vi "AeroQuadConfigurator.vi"() -> ()   [LabVIEW 2009] (continued)
                  n217 = local write "DerivativePitchLevel"(w359) -> ()
                }
                frame #5 {
                  n218 = Index Array(array=w365) -> (element #1=w367:dbl, element #2=w366:dbl)  [unwired: 2 in]
                  n219 = local write "Level Limit"(w367) -> ()
                  n220 = local write "Level Off"(w366) -> ()
                }
                frame #6 {
                  n221 = Index Array(array=w374) -> (element #1=w373:dbl, element #2=w372:dbl, element #3=w371:dbl, element #4=w370:dbl, element #5=w369:dbl, element #6=w368:dbl)  [unwired: 6 in]
                  n222 = local write "Roll Smoothing"(w373) -> ()
                  n223 = local write "Pitch Smoothing"(w372) -> ()
                  n224 = local write "Yaw  Smoothing"(w371) -> ()
                  n225 = local write "Throttle Smoothing"(w370) -> ()
                  n226 = local write "Mode  Smoothing"(w369) -> ()
                  n227 = local write "Aux  Smoothing"(w368) -> ()
                }
              }
            }
            n228 = local write "Status"("Reading Configuration" ("Connection Status")) -> ()
            n229 = Bundle By Name(cluster=w320, "Error"=w311) -> (w321:T11)
          }
        }
      }
      frame #18 {
        n230 = Unbundle By Name(w378) -> ("Connected"=w376:bool, "COMport"=w379:refnum<visa-resource-name>)
        n231 = case shown="True" w376 {
          tunnel: w379 -> [_ w392]
          tunnel: w378 -> [w380 w390]
          tunnel: [w380 w389] -> w377
          tunnel: w375 -> [_ w385]
          frame #0 {
          }
          frame #1 {
            n232 = Flush Queue(queue=w385) -> (queue out=w387:refnum<queue>)  [unwired: 1 in, 2 out]
            n233 = property on="PID / Sensor Output" class="WFChart (strict)"("History Data"=cluster{"[0]":i16, "[1]":i16, "[2]":i16}[] []) -> ()  [unwired: 2 in, 2 out]
            n234 = VISA Write(VISA resource name=w392, write buffer="S") -> (error out=w388:errorcluster)  [unwired: 1 in, 2 out]
            n235 = Bundle By Name(cluster=w390, "Error"=w388) -> (w389:T11)
            n236 = property on="Motor Commands" class="WFChart (strict)"("History Data"=T9 []) -> ()  [unwired: 2 in, 2 out]
            n237 = Enqueue Element(queue=w387, element="Read AeroQuad Data") -> (queue out=w384:refnum<queue>)  [unwired: 1 in, 3 out]
            n238 = Enqueue Element(queue=w384, element="Status:Reading Flight Data") -> ()  [unwired: 1 in, 4 out]
          }
        }
      }
      frame #19 {
        n239 = Unbundle By Name(w405) -> ("Connected"=w402:bool, "COMport"=w406:refnum<visa-resource-name>, "Timeout"=w393:u32)
        n240 = Spreadsheet String To Array(delimiter (Tab)=",", format string="%s", spreadsheet string=w400, array type (2D Dbl)=string[] []) -> (array=w396:string[])
        n241 = Build Array (concatenate)("a0;", w396) -> (w394:string[])
        n242 = case shown="True" w402 {
          tunnel: w406 -> [_ w412]
          tunnel: [w409 w415] -> w404
          tunnel: w394 -> [_ w414]
          tunnel: w401 -> [w408 _]
          tunnel: w393 -> [_ w410]
          frame #0 {
            n243 = local write "Status"("Not Connected to AeroQuad" ("Connection Status")) -> ()
            n244 = Flush Queue(queue=w408) -> (error out=w409:errorcluster)  [unwired: 1 in, 2 out]
          }
          frame #1 {
            n245 = property class="Instr"(reference=w412, "Timeout"=w410) -> (reference out=w413:refnum<visa-resource-name>, error out=w411:errorcluster)  [unwired: 1 in]
            n246 = VISA Write(VISA resource name=w413, write buffer="X", error in (no error)=w411) -> (VISA resource name out=w418:refnum<visa-resource-name>, error out=w420:errorcluster)  [unwired: 1 out]
            n247 = call "Time Delay18"("error in (no error)"=w420) -> ("error out"=w419:errorcluster)  [unwired: 1 in, 9 out]
            n248 = VISA Flush I/O Buffer(VISA resource name=w418, error in (no error)=w419) -> (VISA resource name out=w416:refnum<visa-resource-name>, error out=w417:errorcluster)  [unwired: 1 in]
            n249 = for {
              tunnel: w416 -> [w424]
              shift-right: [w423] -> w415
              shift-left: w417 -> [w425]
              tunnel: w414 -> [w422] mode=indexing
              n250 = VISA Write(VISA resource name=w424, write buffer=w422, error in (no error)=w425) -> (error out=w423:errorcluster)  [unwired: 2 out]
            }
          }
        }
        n251 = Bundle By Name(cluster=w405, "Error"=w404) -> (w403:T11)
      }
      frame #20 {
        n252 = Unbundle By Name(w431) -> ("Connected"=w428:bool, "COMport"=w432:refnum<visa-resource-name>)
        n253 = case shown="True" w428 {
          tunnel: w432 -> [_ w448]
          tunnel: [w435 w439] -> w430
          tunnel: w426 -> [_ w437]
          tunnel: w427 -> [w434 w445]
          frame #0 {
            n254 = local write "Status"("Not Connected to AeroQuad" ("Connection Status")) -> ()
            n255 = Flush Queue(queue=w434) -> (error out=w435:errorcluster)  [unwired: 1 in, 2 out]
          }
          frame #1 {
            n256 = VISA Write(VISA resource name=w448, write buffer="X") -> (VISA resource name out=w449:refnum<visa-resource-name>, error out=w451:errorcluster)  [unwired: 1 in, 1 out]
            n257 = call "Time Delay9"("error in (no error)"=w451) -> ("error out"=w450:errorcluster)  [unwired: 1 in, 9 out]
            n258 = VISA Flush I/O Buffer(VISA resource name=w449, error in (no error)=w450) -> (VISA resource name out=w446:refnum<visa-resource-name>, error out=w447:errorcluster)  [unwired: 1 in]
            n259 = Concatenate Strings("a0;" ("string"), w437) -> (w438:string)
            n260 = VISA Write(VISA resource name=w446, write buffer=w438, error in (no error)=w447) -> (VISA resource name out=w440:refnum<visa-resource-name>, error out=w442:errorcluster)  [unwired: 1 out]
            n261 = property class="Instr"(reference=w440, error in=w442, "General Settings:Timeout Value"=u32 500) -> (error out=w441:errorcluster)  [unwired: 1 out]
            n262 = Enqueue Element(queue=w445, element="Read Serial Monitor Data", error in (no error)=w441) -> (error out=w439:errorcluster)  [unwired: 3 out]
          }
        }
        n263 = Bundle By Name(cluster=w431, "Error"=w430) -> (w429:T11)
      }
      frame #21 {
        w453 = T8."Disabled and Grayed Out" ("Disabled")
        n264 = Unbundle By Name(w465) -> ("COMport"=w461:refnum<visa-resource-name>)
        n265 = VISA Flush I/O Buffer(VISA resource name=w461) -> (VISA resource name out=w460:refnum<visa-resource-name>, error out=w462:errorcluster)  [unwired: 2 in]
        n266 = Enqueue Element(queue=w455, element="Status:Disconnected from AeroQuad") -> ()  [unwired: 1 in, 4 out]
        n267 = call "Time Delay7"("error in (no error)"=w462) -> ("error out"=w459:errorcluster)  [unwired: 1 in, 9 out]
        n268 = VISA Close(VISA resource name=w460, error in (no error)=w459) -> (error out=w458:errorcluster)
        n269 = call <vilib>:"Clear Errors.vi"("error in (no error)"=w458) -> ("error out"=w457:errorcluster)  [unwired: 6 out]
        n270 = Bundle By Name(cluster=w465, "Connected"=FALSE, "Error"=w457) -> (w464:T11)
        n271 = property on="Connect" class="Bool"("Disabled"=T8."Enabled") -> ()  [unwired: 2 in, 2 out]
        n272 = property on="SendCommand" class="Bool"("DisabledEnum"=w453) -> ()  [unwired: 2 in, 2 out]
        n273 = property on="Disconnect" class="Bool"("Disabled"=w453) -> ()  [unwired: 2 in, 2 out]
        n274 = property on="PerformPreFlightCheckout" class="Bool"("Disabled"=w453) -> ()  [unwired: 2 in, 2 out]
        n275 = property on="InitializeEEPROM" class="Bool"("Disabled"=w453) -> ()  [unwired: 2 in, 2 out]
        n276 = property on="SaveFlightData" class="Bool (strict)"("DisabledEnum"=w453) -> ()  [unwired: 2 in, 2 out]
        n277 = property on="CalibrateTransmitterFront" class="Bool"("Disabled"=w453) -> ()  [unwired: 2 in, 2 out]
        n278 = property on="CalibrateTransmitter" class="Bool"("Disabled"=w453) -> ()  [unwired: 2 in, 2 out]
        n279 = property on="CalibrateESCs" class="Bool"("Disabled"=w453) -> ()  [unwired: 2 in, 2 out]
        n280 = property on="DefaultTransmitterValue" class="Bool"("Disabled"=w453) -> ()  [unwired: 2 in, 2 out]
        n281 = property on="UpdateXmit" class="Bool"("DisabledEnum"=w453) -> ()  [unwired: 2 in, 2 out]
        n282 = property on="UpdateAcro" class="Bool"("DisabledEnum"=w453) -> ()  [unwired: 2 in, 2 out]
        n283 = property on="UpdateSensors" class="Bool"("DisabledEnum"=w453) -> ()  [unwired: 2 in, 2 out]
        n284 = property on="UpdateStable" class="Bool"("DisabledEnum"=w453) -> ()  [unwired: 2 in, 2 out]
        n285 = property on="UpdateXmit" class="Bool"("DisabledEnum"=w453) -> ()  [unwired: 2 in, 2 out]
        n286 = property on="CalibrateGyros" class="Bool"("DisabledEnum"=w453) -> ()  [unwired: 2 in, 2 out]
        n287 = property on="CalibrateAccels" class="Bool"("DisabledEnum"=w453) -> ()  [unwired: 2 in, 2 out]
        n288 = property on="SendMotorCommand" class="Bool"("DisabledEnum"=w453) -> ()  [unwired: 2 in, 2 out]
      }
      frame #22 {
        n289 = Unbundle By Name(w470) -> ("Error"=w469:errorcluster)
        n290 = call "ReconnectDialog.vi"("error in"=w469) -> ("error out"=w468:errorcluster, "AbortConnection"=w466:bool)  [unwired: 9 out]
        n291 = case shown="True" w466 {
          tunnel: w468 -> [_ _]
          tunnel: w467 -> [w472 _]
          frame #0 {
            n292 = Flush Queue(queue=w472) -> (queue out=w471:refnum<queue>)  [unwired: 1 in, 2 out]
            n293 = Enqueue Element(queue=w471, element="Open COM Port") -> ()  [unwired: 1 in, 4 out]
          }
          frame #1 {
            n294 = local write "GUI"(0) -> ()
          }
        }
      }
      frame #23 {
      }
      frame #24 {
        n295 = Enqueue Element(queue=w486, element="Command:O1;0;1;0;1;0;1;0;1;0;1;0;,U") -> (queue out=w484:refnum<queue>)  [unwired: 1 in, 3 out]
        n296 = Enqueue Element(queue=w484, element="Read Transmitter Data") -> ()  [unwired: 1 in, 4 out]
        n297 = Initialize Array(i16 -32768 ("ThrottleMin"), 6 ("dimension size")) -> (w477:i16[])
        n298 = Initialize Array(i16 32767 ("ThrottleMin"), 6 ("dimension size")) -> (w478:i16[])
        n299 = Bundle By Name(cluster=w488, "MaxLimits"=w477, "MinLimits"=w478) -> (w487:T11)
        n300 = local write "Status"("Transmitter Calibration Values Initialized" ("Connection Status")) -> ()
      }
      frame #25 {
        n301 = Unbundle By Name(w499) -> ("MaxLimits"=w495:i16[], "MinLimits"=w494:i16[], "COMport"=w497:refnum<visa-resource-name>)
        n302 = Subtract(x=w495, y=w494) -> (x-y=w493:i16[])
        n303 = Greater Or Equal?(x=w493, y=i16 500) -> (x >= y?=w490:bool[])
        n304 = And Array Elements(Boolean array=w490) -> (logical AND=w491:bool)
        n305 = case shown="True" w491 {
          tunnel: w494 -> [_ w550]
          tunnel: w495 -> [_ w549]
          tunnel: w497 -> [w501 w542]
          tunnel: [w500 w535] -> w496
          tunnel: w490 -> [w506 _]
          tunnel: w489 -> [w513 w540]
          frame #0 {
            n306 = Flush Queue(queue=w513) -> (queue out=w514:refnum<queue>)  [unwired: 1 in, 2 out]
            n307 = VISA Write(VISA resource name=w501, write buffer="X") -> (VISA resource name out=w502:refnum<visa-resource-name>, error out=w504:errorcluster)  [unwired: 1 in, 1 out]
            n308 = call "Time Delay3"("error in (no error)"=w504) -> ("error out"=w503:errorcluster)  [unwired: 1 in, 9 out]
            n309 = VISA Flush I/O Buffer(VISA resource name=w502, error in (no error)=w503) -> (error out=w500:errorcluster)  [unwired: 1 in, 1 out]
            n310 = for {
              tunnel: w506 -> [w523] mode=indexing
              shift-right: [w520] -> w517
              shift-left: "" -> [w521]
              tunnel: string[] ["Roll", "Pitch", "Yaw", "Throttle", "Mode", "Aux"] -> [w522] mode=indexing
              n311 = case shown="False" w523 {
                tunnel: w522 -> [w525 _]
                tunnel: [w527 w528] -> w520
                tunnel: w521 -> [w526 w528]
                frame #0 {
                  n312 = Concatenate Strings(w526, w525, "\r\n") -> (w527:string)
                }
                frame #1 {
                }
              }
            }
            n313 = Enqueue Element(queue=w514, element="Status: Transmitter NOT Calibrated") -> (queue out=w515:refnum<queue>)  [unwired: 1 in, 3 out]
            n314 = Format Into String(format string="Dialog:The following channels appear NOT to be calibrated:\n\n%s\nPlease be sure to move all transmitter sticks and flip all switches when performing the transmitter calibration.", w517) -> (resulting string=w507:string)  [unwired: 2 in, 1 out]
            n315 = Enqueue Element(queue=w515, element=w507) -> (queue out=w509:refnum<queue>)  [unwired: 1 in, 3 out]
            n316 = Enqueue Element(queue=w509, element="Command:U") -> (queue out=w511:refnum<queue>)  [unwired: 1 in, 3 out]
            n317 = Enqueue Element(queue=w511, element="Read Transmitter Data") -> ()  [unwired: 1 in, 4 out]
          }
          frame #1 {
            # "y = mx + b\n\nm = (y2 - y1) / (x2 - x1)\n    = (2000 - 1000) / (TxMax - TxMin)\n    = 1000 / (TxMax - TxMin)\n\nb = y1 - m(x1)\n   = 1000 - m(TxMin)"
            n318 = for {
              tunnel: w550 -> [w554] mode=indexing
              tunnel: w549 -> [w559] mode=indexing
              tunnel: [w553] -> w548 mode=indexing
              tunnel: [w551] -> w547 mode=indexing
              # "b"
              # "m"
              n319 = Subtract(x=w559, y=w554) -> (x-y=w558:i16)
              n320 = To Double Precision Float(number=w558) -> (double precision float=w557:dbl)
              n321 = To Double Precision Float(number=w554) -> (double precision float=w552:dbl)
              n322 = Divide(x=1000.0, y=w557) -> (x/y=w553:dbl)
              n323 = Multiply(x=w552, y=w553) -> (x*y=w555:dbl)
              n324 = Subtract(x=1000.0, y=w555) -> (x-y=w551:dbl)
            }
            n325 = VISA Write(VISA resource name=w542, write buffer="X") -> (VISA resource name out=w543:refnum<visa-resource-name>, error out=w545:errorcluster)  [unwired: 1 in, 1 out]
            n326 = call "Time Delay8"("error in (no error)"=w545) -> ("error out"=w544:errorcluster)  [unwired: 1 in, 9 out]
            n327 = VISA Flush I/O Buffer(VISA resource name=w543, error in (no error)=w544) -> (VISA resource name out=w537:refnum<visa-resource-name>, error out=w536:errorcluster)  [unwired: 1 in]
            n328 = Enqueue Element At Opposite End(queue=w540, element="Status:Transmitter Calibration Values Saved" ("Connection Status")) -> ()  [unwired: 1 in, 4 out]
            n329 = Interleave 1D Arrays(w548, w547) -> (w532:dbl[])
            n330 = Number To Fractional String(number=w532, precision (6)=i16 2) -> (F-format string=w530:string[])  [unwired: 2 out]
            n331 = Fract/Exp String To Number(string=w530) -> (number=w529:dbl[])  [unwired: 4 out]
            n332 = call "WriteEEPROM.vi"("Write Data to EEPROM"=TRUE, "Query"="P", "Data"=w529, "Command"="O", "error in"=w536, "Skip"=TRUE, "VISA resource name"=w537) -> ("error out"=w535:errorcluster)  [unwired: 4 out]
          }
        }
        n333 = Bundle By Name(cluster=w499, "Error"=w496) -> (w498:T11)
      }
      frame #26 {
        n334 = Unbundle By Name(w565) -> ("COMport"=w569:refnum<visa-resource-name>)
        n335 = flat-sequence {
          tunnel: w569 -> [w615]
          tunnel: [w614] -> w568
          tunnel: [w613] -> w567
          tunnel: w568 -> [w625]
          tunnel: w567 -> [w626]
          tunnel: [w623] -> w563
          tunnel: [w622] -> w562
          tunnel: [w621] -> w561
          frame #0 {
            n336 = local write "Status"("Calibrating ESC's" ("Connection Status")) -> ()
            n337 = VISA Write(VISA resource name=w615, write buffer="X") -> (VISA resource name out=w618:refnum<visa-resource-name>, error out=w616:errorcluster)  [unwired: 1 in, 1 out]
            n338 = call "Time Delay14"("error in (no error)"=w616) -> ("error out"=w617:errorcluster)  [unwired: 1 in, 9 out]
            n339 = VISA Flush I/O Buffer(VISA resource name=w618, error in (no error)=w617) -> (VISA resource name out=w613:refnum<visa-resource-name>, error out=w614:errorcluster)  [unwired: 1 in]
          }
          frame #1 {
            n340 = VISA Write(VISA resource name=w626, write buffer="1", error in (no error)=w625) -> (VISA resource name out=w622:refnum<visa-resource-name>, error out=w623:errorcluster)  [unwired: 1 out]
            n341 = Two Button Dialog(message="This calibration process is for the Turnigy ESC's only.  This may work with other ESC's, consult the manufacturer's manual.\n\nWarning! Before starting this calibration, be sure to securely hold down the quad or remove the propellers for safety considerations!\n\nWhat to expect: You should hear 2 short beeps when the high throttle position is being calibrated.  Then you wll hear 3 short beeps followed by1 long beep once the low throttle position is calibrated.\n\nApply power to the ESC's and motors, then quickly hit OK.", 1:"Abort" ("F button name (\"Cancel\")")) -> (T button?=w621:bool)  [unwired: 1 out]
          }
        }
        n342 = case shown="True" w561 {
          tunnel: [w570 w579] -> w566
          tunnel: w563 -> [w571 w578]
          tunnel: w562 -> [w572 w576]
          frame #0 {
            n343 = local write "Status"("ESC Calibration Aborted" ("Connection Status")) -> ()
            n344 = VISA Write(VISA resource name=w572, write buffer="4", error in (no error)=w571) -> (error out=w570:errorcluster)  [unwired: 2 out]
          }
          frame #1 {
            n345 = flat-sequence {
              tunnel: [w587] -> w584
              tunnel: w578 -> [w586]
              tunnel: [w585] -> w577
              tunnel: w576 -> [w585]
              tunnel: [w593] -> w583
              tunnel: [w592] -> w582
              tunnel: w584 -> [w591]
              tunnel: w577 -> [w590]
              tunnel: [w601] -> w581
              tunnel: [w600] -> w580
              tunnel: w583 -> [w598]
              tunnel: w582 -> [w599]
              tunnel: w581 -> [w607]
              tunnel: w580 -> [w606]
              tunnel: [w608] -> w575
              tunnel: [w612] -> w579
              tunnel: w575 -> [w612]
              frame #0 {
                n346 = local write "Status"("Calibrating High Throttle" ("Connection Status")) -> ()
                n347 = call "Time Delay15"("error in (no error)"=w586, "Delay Time (s)"=2.0) -> ("error out"=w587:errorcluster)  [unwired: 9 out]
              }
              frame #1 {
                n348 = VISA Write(VISA resource name=w590, write buffer="2", error in (no error)=w591) -> (VISA resource name out=w593:refnum<visa-resource-name>, error out=w595:errorcluster)  [unwired: 1 out]
                n349 = local write "Status"("Calibrating Low Throttle" ("Connection Status")) -> ()
                n350 = call "Time Delay16"("error in (no error)"=w595, "Delay Time (s)"=4.0) -> ("error out"=w592:errorcluster)  [unwired: 9 out]
              }
              frame #2 {
                n351 = Format Into String(format string="3%d;", "Minimum Test Throttle") -> (resulting string=w605:string)  [unwired: 2 in, 1 out]
                n352 = VISA Write(VISA resource name=w598, write buffer=w605, error in (no error)=w599) -> (VISA resource name out=w600:refnum<visa-resource-name>, error out=w601:errorcluster)  [unwired: 1 out]
                n353 = One Button Dialog(message="Are all the motors spinning at the same rate?  If not, perform the calibration again.") -> ()  [unwired: 2 out]
              }
              frame #3 {
                n354 = local write "Status"("ESC Calibration Complete" ("Connection Status")) -> ()
                n355 = VISA Write(VISA resource name=w606, write buffer="4", error in (no error)=w607) -> (error out=w608:errorcluster)  [unwired: 2 out]
              }
              frame #4 {
                w611 = 4
                n356 = local write "PlotSelection"(w611) -> ()
                n357 = local write "GUI"(w611) -> ()
              }
            }
          }
        }
        n358 = Bundle By Name(cluster=w565, "Error"=w566) -> (w564:T11)
      }
      frame #27 {
        n359 = Initialize Array(i16 2000, 6 ("dimension size")) -> (w629:i16[])
        n360 = Initialize Array(i16 1000, 6 ("dimension size")) -> (w630:i16[])
        n361 = Bundle By Name(cluster=w636, "MaxLimits"=w629, "MinLimits"=w630) -> (w635:T11)
      }
      frame #28 {
      }
      frame #29 {
        n362 = Unbundle By Name(w677) -> ("COMport"=w644:refnum<visa-resource-name>, "Output Type"=w650:T4, "Motor Plot"=w645:enum16{"Motor Chart", "Motor Bar Plot"})
        n363 = VISA Read(VISA resource name=w644, byte count=u32 1024) -> (read buffer=w659:string, error out=w658:errorcluster)  [unwired: 1 in, 2 out]
        n364 = Enqueue Element(queue=w671, element="Read AeroQuad Data") -> (queue out=w642:refnum<queue>)  [unwired: 1 in, 3 out]
        n365 = Bundle By Name(cluster=w677, "Error"=w658) -> (w676:T11)
        n366 = Spreadsheet String To Array(delimiter (Tab)=",", format string="%s", spreadsheet string=w659, array type (2D Dbl)=i16[] [0]) -> (array=w670:i16[])
        n367 = Split 1D Array(array=w670, index=1) -> (first subarray=w647:i16[], second subarray=w668:i16[])
        n368 = Split 1D Array(array=w668, index=3) -> (first subarray=w657:i16[], second subarray=w667:i16[])
        n369 = Split 1D Array(array=w667, index=4) -> (first subarray=w648:i16[], second subarray=w665:i16[])
        n370 = Index Array(array=w647) -> (element=→"Loop Rate":i16)  [unwired: 1 in]
        n371 = Split 1D Array(array=w665, index=4) -> (first subarray=w661:i16[], second subarray=w655:i16[])
        n372 = Enqueue Element(queue=w642, element="Status:Reading Flight Data") -> ()  [unwired: 1 in, 4 out]
        n373 = Index Array(array=w655) -> (element #1=w649:i16, element #2=w653:i16)  [unwired: 2 in]
        n374 = Index Array(array=w657) -> (element #1=→"Roll":i16, element #2=w662:i16, element #3=→"Yaw":i16)  [unwired: 3 in]
        n375 = Not Equal To 0?(x=w649) -> (x != 0?=→"Armed":bool)
        n376 = case shown="\"PID Chart\"" w650 {
          tunnel: w657 -> [w685 _]
          tunnel: [w685 w686] -> w656
          tunnel: w648 -> [_ w687]
          frame #0 {
          }
          frame #1 {
            n377 = Split 1D Array(array=w687, index=1) -> (second subarray=w686:i16[])  [unwired: 1 out]
          }
        }
        n378 = Negate(x=w662) -> (-x=→"Pitch":i16)
        n379 = Less?(x=w653, y=i16 1500) -> (x < y?=→"Mode 2":bool)
        n380 = Array To Cluster(array=w656) -> (cluster=→"PID / Sensor Output":cluster{"[0]":i16, "[1]":i16, "[2]":i16})
        n381 = case shown="\"Motor Chart\", Default" w645 {
          tunnel: w661 -> [w679 w684]
          frame #0 {
            n382 = Array To Cluster(array=w679) -> (cluster=→"Motor Commands":T3)
          }
          frame #1 {
            n383 = Index Array(array=w684) -> (element #1=→"Front Motor":i16, element #2=→"Rear Motor":i16, element #3=→"Right Motor":i16, element #4=→"Left Motor":i16)  [unwired: 4 in]
          }
        }
      }
      frame #30 {
        n384 = Unbundle By Name(w713) -> ("CurrentTime"=w698:timestamp, "dT"=w699:dbl, "DataRef"=w703:refnum<k34>, "Save"=w704:bool, "COMport"=w714:refnum<visa-resource-name>)
        n385 = Enqueue Element(queue=w706, element="Read Sensor Data") -> (queue out=w697:refnum<queue>)  [unwired: 1 in, 3 out]
        n386 = VISA Read(VISA resource name=w714, byte count=u32 1024) -> (read buffer=w716:string, error out=w702:errorcluster)  [unwired: 1 in, 2 out]
        n387 = Spreadsheet String To Array(delimiter (Tab)=",", format string="%s", spreadsheet string=w716, array type (2D Dbl)=dbl[] [0.0]) -> (array=w692:dbl[])
        n388 = case shown="True" w704 {
          tunnel: w692 -> [_ w725]
          tunnel: w703 -> [_ w734]
          tunnel: w702 -> [w721 w736]
          tunnel: [w721 w735] -> w701
          tunnel: [0.0 w730] -> w700
          tunnel: w699 -> [_ w733]
          tunnel: w698 -> [_ w731]
          frame #0 {
          }
          frame #1 {
            n389 = Delete From Array(array=w725, length=2, index=6) -> (array with subset deleted=w726:dbl[])  [unwired: 1 out]
            n390 = Add(x=0.1, y=w733) -> (x+y=w730:dbl)
            n391 = for {
              tunnel: w726 -> [w740] mode=indexing
              tunnel: w731 -> [w737]
              tunnel: w730 -> [w738]
              tunnel: dbl[] [0.0] -> [w742]
              tunnel: [w741] -> w728 mode=indexing
              n392 = Replace Array Subset(array=w742, new element=w740) -> (w739:dbl[])  [unwired: 1 in]
              n393 = Bundle By Name("t0"=w737, "Y"=w739, "dt"=w738) -> (w741:waveform(dbl))  [unwired: 1 out]
            }
            n394 = TDMS Write(0:w734, 5:"AeroQuad Sensor Data", 7:string[] ["Roll Gyro ADC", "Pitch Gyro ADC", "Yaw Gyro ADC", "Roll Accel ADC", "Pitch Accel ADC", "Z Axis Accel ADC", "Roll Flight Angle", "Pitch Flight Angle"] ("channel name(s) in (Untitled)"), 9:w728, 11:w736) -> (15:w735:errorcluster)  [unwired: 1 in, 3 out]
          }
        }
        n395 = Enqueue Element(queue=w697, element="Status:Reading Sensor Data") -> ()  [unwired: 1 in, 4 out]
        n396 = Array To Cluster(array=w692) -> (cluster=→"Raw Data":T5)
        n397 = Index Array(array=w692, index #1=6 ("index")) -> (element #1=w693:dbl, element #2=w694:dbl, element #3=w708:dbl, element #4=w707:dbl)  [unwired: 3 in]
        n398 = Index Array(array=w692, index #1=8 ("index")) -> (element #1=→"Roll Angle":dbl, element #2=→"Pitch Angle":dbl)  [unwired: 1 in]
        n399 = Bundle(w708, w693) -> (→"Auto Level Roll":cluster{dbl, dbl})  [unwired: 1 out]
        n400 = Bundle(w707, w694) -> (→"Auto Level Pitch":cluster{dbl, dbl})  [unwired: 1 out]
        n401 = Bundle By Name(cluster=w713, "dT"=w700, "Error"=w701) -> (w712:T11)
      }
      frame #31 {
        n402 = Unbundle By Name(w749) -> ("COMport"=w756:refnum<visa-resource-name>)
        n403 = Enqueue Element(queue=w759, element="Read Yaw Data") -> (queue out=w761:refnum<queue>)  [unwired: 1 in, 3 out]
        n404 = VISA Read(VISA resource name=w756, byte count=u32 1024) -> (read buffer=w752:string, error out=w747:errorcluster)  [unwired: 1 in, 2 out]
        n405 = Bundle By Name(cluster=w749, "Error"=w747) -> (w748:T11)
        n406 = Spreadsheet String To Array(delimiter (Tab)=",", format string="%s", spreadsheet string=w752, array type (2D Dbl)=dbl[] [0.0]) -> (array=w751:dbl[])
        n407 = Enqueue Element(queue=w761, element="Status:Reading Current Heading") -> ()  [unwired: 1 in, 4 out]
        n408 = Index Array(array=w751) -> (element #1=→"Transmitter Yaw Command":dbl, element #2=→"Delta Heading" →"DeltaHeading":dbl, element #3=w745:dbl, element #4=w746:dbl)  [unwired: 4 in]
        n409 = Bundle(w745, w746) -> (→"Heading":cluster{dbl, dbl})  [unwired: 1 in]
      }
      frame #32 {
        n410 = Unbundle By Name(w773) -> ("MaxLimits"=w767:i16[], "MinLimits"=w768:i16[], "COMport"=w774:refnum<visa-resource-name>)
        n411 = Enqueue Element(queue=w770, element="Read Transmitter Data") -> (queue out=w762:refnum<queue>)  [unwired: 1 in, 3 out]
        n412 = VISA Read(VISA resource name=w774, byte count=u32 1024) -> (read buffer=w776:string, error out=w771:errorcluster)  [unwired: 1 in, 2 out]
        n413 = Spreadsheet String To Array(delimiter (Tab)=",", format string="%s", spreadsheet string=w776, array type (2D Dbl)=i16[] [0]) -> (array=w764:i16[])
        n414 = for {
          tunnel: w768 -> [w786] mode=indexing
          tunnel: w764 -> [w780] mode=indexing
          tunnel: w767 -> [w785] mode=indexing
          tunnel: [w784] -> w766 mode=indexing
          tunnel: [w781] -> w765 mode=indexing
          i -> [w783]
          n415 = Max & Min(x=w785, y=w780) -> (max(x,y)=w781:i16)  [unwired: 1 out]
          n416 = Max & Min(x=w786, y=w780) -> (min(x,y)=w784:i16)  [unwired: 1 out]
          n417 = Bundle(w781, w784, w780) -> (w782:cluster{i16, i16, i16})  [unwired: 1 out]
          n418 = case shown="5" w783 {
            tunnel: w782 -> [w787 w788 w789 w790 w791 w792]
            frame #0 {
              "Roll Channel" <- w787
            }
            frame #1 {
              "Pitch Channel" <- w788
            }
            frame #2 {
              "Yaw Channel" <- w789
            }
            frame #3 {
              "Throttle Channel" <- w790
            }
            frame #4 {
              "Mode" <- w791
            }
            frame #5 {
              "Aux" <- w792
            }
          }
        }
        n419 = Enqueue Element(queue=w762, element="Status:Reading Transmitter Data") -> ()  [unwired: 1 in, 4 out]
        n420 = Bundle By Name(cluster=w773, "MaxLimits"=w765, "MinLimits"=w766, "Error"=w771) -> (w772:T11)
      }
      frame #33 {
        n421 = Unbundle By Name(w805) -> ("COMport"=w807:refnum<visa-resource-name>)
        n422 = Enqueue Element(queue=w803, element="Read Command Data") -> (queue out=w794:refnum<queue>)  [unwired: 1 in, 3 out]
        n423 = VISA Read(VISA resource name=w807, byte count=u32 1024) -> (read buffer=w809:string, error out=w806:errorcluster)  [unwired: 1 in, 2 out]
        n424 = Spreadsheet String To Array(delimiter (Tab)=",", format string="%s", spreadsheet string=w809, array type (2D Dbl)=dbl[] [0.0]) -> (array=w801:dbl[])
        n425 = Enqueue Element(queue=w794, element="Status:Reading Command Data") -> ()  [unwired: 1 in, 4 out]
        n426 = Bundle By Name(cluster=w805, "Error"=w806) -> (w804:T11)
        n427 = Split 1D Array(array=w801, index=1) -> (first subarray=w798:dbl[], second subarray=w799:dbl[])
        n428 = Index Array(array=w798) -> (element=→"Transmitter Factor Indicator":dbl)  [unwired: 1 in]
        n429 = To Word Integer(number=w799) -> (16bit integer=w796:i16[])
        n430 = Array To Cluster(array=w796) -> (cluster=→"Command Data":T6)
      }
      frame #34 {
        n431 = Unbundle By Name(w826) -> ("COMport"=w813:refnum<visa-resource-name>)
        n432 = property on="SerialData" class="Str"() -> ("Value"=w823:string)  [unwired: 2 in, 2 out]
        n433 = VISA Read(VISA resource name=w813, byte count=u32 1024) -> (read buffer=w824:string, error out=w818:errorcluster)  [unwired: 1 in, 2 out]
        n434 = Concatenate Strings(w823, w824) -> (w820:string)
        n435 = feedback #1(0) -> (w821:i32)
        n436 = Increment(x=w821) -> (x+1=w815:i32)
        n437 = property on="SerialData" class="Str"("Value"=w820, "Text.Scroll Position"=w815) -> ()  [unwired: 2 in, 2 out]
        n438 = case shown="128.." w815 {
          selector: w815 -> [w835 _]
          tunnel: [w835 0] -> w819
          frame #0 {
          }
          frame #1 {
            "SerialData" <- ""
          }
        }
        n439 = Unbundle By Name(w818) -> ("code"=w817:i32)
        n440 = case shown="0" w817 {
          tunnel: w818 -> [w828 w830 w833]
          tunnel: [w828 w829 w832] -> w814
          tunnel: w816 -> [_ _ w834]
          frame #0 {
          }
          frame #1 {
            n441 = call <vilib>:"Clear Errors.vi"("error in (no error)"=w830) -> ("error out"=w829:errorcluster)  [unwired: 6 in]
          }
          frame #2 {
            n442 = Enqueue Element(queue=w834, element="Read Serial Monitor Data", error in (no error)=w833) -> (error out=w832:errorcluster)  [unwired: 3 out]
          }
        }
        n443 = Bundle By Name(cluster=w826, "Error"=w814) -> (w825:T11)
      }
      frame #35 {
        # "12 byte string\n(2 bytes = int)\n\nRoll Gyro\nPitch Gyro\nYaw Gyro\nRoll Acc\nPitch Acc\nZ Acc"
        n444 = Unbundle By Name(w839) -> ("AREF"=w838:dbl)
        n445 = Unbundle By Name(w839) -> ("ResetFFT"=w840:bool, "COMport"=w842:refnum<visa-resource-name>, "Connected"=w845:bool)
        n446 = case shown="True" w845 {
          tunnel: w842 -> [_ w859]
          tunnel: w839 -> [w846 w861]
          tunnel: [w846 w860] -> w841
          tunnel: w840 -> [_ w850]
          tunnel: w838 -> [_ w847]
          frame #0 {
          }
          frame #1 {
            w855 = 0 items=["no exception", "cancel error on match", "set error on match"] ("[exception action] (none:0)")
            w856 = T14 0 items=["no dialog", "OK message", "continue or stop message", "OK message + warnings", "continue/stop + warnings"] ("type of dialog (OK msg:1)")
            n447 = call "DecodeSensorBytes.vi"("VISA resource name"=w859) -> ("error out"=w857:errorcluster, "Array"=w858:i16[][], "Bytes"=→"Bytes To Process":u32)  [unwired: 7 in, 1 out]
            n448 = Compound Arithmetic op=OR("ResetFFT", w850) -> (w849:bool)
            n449 = for {
              tunnel: w858 -> [w876] mode=indexing
              tunnel: w847 -> [w872]
              tunnel: w849 -> [w863]
              n450 = Index Array(array=w876, index="Signal") -> (element=w864:i16)
              "Time Domain" <- w864
              n451 = Multiply(x=w872, y=w864) -> (x*y=w865:dbl)
              n452 = call <vilib>:"Auto Power Spectrum PtByPt.vi"("signal"=w865, "sample length"=512, "dt"=0.01, "initialize"=w863) -> ("Power Spectrum (V^2 rms)"=w875:dbl[], "df"=w879:dbl)  [unwired: 1 in, 1 out]
              n453 = Array Max & Min(array=w875) -> (max value=w869:dbl, max index (indices)=w873:i32)  [unwired: 2 out]
              n454 = Bundle(0.0, "df"=w879, "Power Spectrum (V^2 rms)"=w875) -> (w871:T7)  [unwired: 1 in]
              n455 = Greater Or Equal?(x=w869, y=1e-06) -> (x >= y?=w867:bool)
              n456 = case shown="True" w867 {
                tunnel: [_ w885] -> w874
                tunnel: w873 -> [_ w884]
                tunnel: [_ w883] -> w870
                tunnel: w871 -> [_ w883]
                tunnel: [TRUE _] -> w866
                frame #0 {
                  n457 = property on="Frequency Domain" class="WFGraph (strict)"("Cursor.Cursor Index"=0) -> ()  [unwired: 2 in, 2 out]
                }
                frame #1 {
                  n458 = property on="Frequency Domain" class="WFGraph (strict)"("Cursor.Cursor Index"=w884) -> ("Cursor.Cursor X"=w885:dbl)  [unwired: 2 in, 2 out]
                }
              }
              "Frequency Domain" <- w870
              "Max Frequency Detected" <- w874
              n459 = property on="NoneFound" class="Str"("Visible"=w866) -> ()  [unwired: 2 in, 2 out]
            }
            n460 = call <vilib>:"General Error Handler.vi"("type of dialog (OK msg:1)"=w856, "error in (no error)"=w857, "[exception action] (none:0)"=w855, "[exception code]"=-1073807252) -> ("error out"=w853:errorcluster)  [unwired: 7 in, 4 out]
            n461 = Bundle By Name(cluster=w861, "ResetFFT"=FALSE, "Error"=w853) -> (w860:T11)
          }
        }
        n462 = Enqueue Element(queue=w843, element="Read Spectrum Analyzer") -> ()  [unwired: 1 in, 4 out]
      }
      frame #36 {
      }
      frame #37 {
        n463 = Unbundle By Name(w893) -> ("COMport"=w888:refnum<visa-resource-name>, "Connected"=w891:bool, "Error"=w890:errorcluster)
        n464 = case shown="True" w891 {
          tunnel: w890 -> [_ w911]
          tunnel: [_ w900] -> w889
          tunnel: w888 -> [_ w912]
          tunnel: "Updating Configuration" ("Connection Status") -> [_ w919]
          frame #0 {
          }
          frame #1 {
            w896 = 0
            n465 = local write "Status"(w919) -> ()
            n466 = VISA Write(VISA resource name=w912, write buffer="X", error in (no error)=w911) -> (VISA resource name out=w915:refnum<visa-resource-name>, error out=w917:errorcluster)  [unwired: 1 out]
            n467 = call "Time Delay5"("error in (no error)"=w917) -> ("error out"=w916:errorcluster)  [unwired: 1 in, 9 out]
            n468 = property on="PlotSelection" class="Ring (strict)"("Value"=w896) -> ()  [unwired: 2 in, 2 out]
            n469 = property on="GUI" class="TabCtl (strict)"("Val(Sgnl)"=w896) -> ()  [unwired: 2 in, 2 out]
            n470 = VISA Flush I/O Buffer(VISA resource name=w915, error in (no error)=w916) -> (VISA resource name out=w914:refnum<visa-resource-name>, error out=w913:errorcluster)  [unwired: 1 in]
            n471 = Build Array("Proportional Roll", "Integral Roll", "Derivative Roll", "ProportionalPitch", "IntegralPitch", "DerivativePitch") -> (w925:dbl[])
            n472 = call "WriteEEPROM.vi"("Query"="B", "Data"=w925, "Command"="A", "error in"=w913, "Skip"=TRUE, "VISA resource name"=w914) -> ("error out"=w898:errorcluster, "Checked Data"=w909:dbl[], "Write Successful"=w895:bool, "VISA resource name out"=w897:refnum<visa-resource-name>)  [unwired: 1 in, 1 out]
            n473 = Index Array(array=w909) -> (element #1=w910:dbl, element #2=w908:dbl, element #3=w907:dbl, element #4=w906:dbl, element #5=w905:dbl, element #6=w904:dbl)  [unwired: 6 in]
            n474 = local read "Transmitter Factor"() -> (w899:dbl)
            n475 = local write "Proportional Roll"(w910) -> ()
            n476 = local write "Integral Roll"(w908) -> ()
            n477 = local write "Derivative Roll"(w907) -> ()
            n478 = local write "ProportionalPitch"(w906) -> ()
            n479 = local write "IntegralPitch"(w905) -> ()
            n480 = local write "DerivativePitch"(w904) -> ()
            n481 = Build Array("Windup Guard", w899) -> (w922:dbl[])
            n482 = call "WriteEEPROM.vi"("Write Data to EEPROM"=TRUE, "Query"="J", "Data"=w922, "Command"="I", "error in"=w898, "Skip"=w895, "VISA resource name"=w897) -> ("error out"=w900:errorcluster, "Checked Data"=w903:dbl[])  [unwired: 3 out]
            n483 = Index Array(array=w903) -> (element #1=w902:dbl, element #2=w901:dbl)  [unwired: 2 in]
            n484 = local write "Windup Guard"(w902) -> ()
            n485 = local write "Transmitter Factor"(w901) -> ()
          }
        }
        n486 = Bundle By Name(cluster=w893, "Error"=w889) -> (w892:T11)
      }
      frame #38 {
        n487 = Unbundle By Name(w936) -> ("COMport"=w937:refnum<visa-resource-name>, "Connected"=w939:bool, "Error"=w938:errorcluster)
        n488 = case shown="True" w939 {
          tunnel: w938 -> [w940 w952]
          tunnel: w937 -> [_ w951]
          tunnel: [w940 w945] -> w935
          frame #0 {
          }
          frame #1 {
            w942 = 1
            n489 = VISA Write(VISA resource name=w951, write buffer="X", error in (no error)=w952) -> (VISA resource name out=w953:refnum<visa-resource-name>, error out=w948:errorcluster)  [unwired: 1 out]
            n490 = call "Time Delay2"() -> ()  [unwired: 2 in, 10 out]
            n491 = VISA Flush I/O Buffer(VISA resource name=w953, error in (no error)=w948) -> (VISA resource name out=w950:refnum<visa-resource-name>, error out=w949:errorcluster)  [unwired: 1 in]
            n492 = property on="GUI" class="TabCtl (strict)"("Val(Sgnl)"=w942) -> ()  [unwired: 2 in, 2 out]
            n493 = property on="PlotSelection" class="Ring (strict)"("Value"=w942) -> ()  [unwired: 2 in, 2 out]
            n494 = Build Array("Gyro Smooth Factor", "Acc Smooth Factor", "Complementary Filter") -> (w959:dbl[])
            n495 = call "WriteEEPROM.vi"("Write Data to EEPROM"=TRUE, "Query"="L", "Data"=w959, "Command"="K", "error in"=w949, "Skip"=TRUE, "VISA resource name"=w950) -> ("error out"=w945:errorcluster, "Checked Data"=w958:dbl[])  [unwired: 3 out]
            n496 = Index Array(array=w958) -> (element #1=w943:dbl, element #2=w957:dbl, element #3=w956:dbl)  [unwired: 3 in]
            n497 = local write "Gyro Smooth Factor"(w943) -> ()
            n498 = local write "Acc Smooth Factor"(w957) -> ()
            n499 = local write "Complementary Filter"(w956) -> ()
            n500 = local write "Status"("Updating Sensor Configuration" ("Connection Status")) -> ()
          }
        }
        n501 = Bundle By Name(cluster=w936, "Error"=w935) -> (w934:T11)
      }
      frame #39 {
        n502 = Unbundle By Name(w965) -> ("COMport"=w966:refnum<visa-resource-name>, "Connected"=w968:bool, "Error"=w967:errorcluster)
        n503 = case shown="True" w968 {
          tunnel: w967 -> [w969 w996]
          tunnel: w966 -> [_ w995]
          tunnel: [w969 w984] -> w964
          frame #0 {
          }
          frame #1 {
            w971 = 3
            n504 = VISA Write(VISA resource name=w995, write buffer="X", error in (no error)=w996) -> (VISA resource name out=w997:refnum<visa-resource-name>, error out=w992:errorcluster)  [unwired: 1 out]
            n505 = call "Time Delay10"() -> ()  [unwired: 2 in, 10 out]
            n506 = local read "Windup Guard"() -> (w990:dbl)
            n507 = VISA Flush I/O Buffer(VISA resource name=w997, error in (no error)=w992) -> (VISA resource name out=w994:refnum<visa-resource-name>, error out=w993:errorcluster)  [unwired: 1 in]
            n508 = property on="GUI" class="TabCtl (strict)"("Val(Sgnl)"=w971) -> ()  [unwired: 2 in, 2 out]
            n509 = property on="PlotSelection" class="Ring (strict)"("Value"=w971) -> ()  [unwired: 2 in, 2 out]
            n510 = Build Array(w990, "Transmitter Factor") -> (w1000:dbl[])
            n511 = call "WriteEEPROM.vi"("Query"="J", "Data"=w1000, "Command"="I", "error in"=w993, "Skip"=TRUE, "VISA resource name"=w994) -> ("error out"=w985:errorcluster, "Checked Data"=w986:dbl[], "Write Successful"=w980:bool, "VISA resource name out"=w981:refnum<visa-resource-name>)  [unwired: 1 in, 1 out]
            n512 = Index Array(array=w986) -> (element #1=w988:dbl, element #2=w987:dbl)  [unwired: 2 in]
            n513 = local write "Windup Guard"(w988) -> ()
            n514 = local write "Transmitter Factor"(w987) -> ()
            n515 = local write "Status"("Updating Transmitter Configuration" ("Connection Status")) -> ()
            n516 = Build Array("Roll Smoothing", "Pitch Smoothing", "Yaw  Smoothing", "Throttle Smoothing", "Mode  Smoothing", "Aux  Smoothing") -> (w973:dbl[])
            n517 = call "WriteEEPROM.vi"("Write Data to EEPROM"=TRUE, "Query"="N", "Data"=w973, "Command"="M", "error in"=w985, "Skip"=w980, "VISA resource name"=w981) -> ("error out"=w984:errorcluster, "Checked Data"=w972:dbl[])  [unwired: 3 out]
            n518 = for {
              tunnel: w972 -> [w1003] mode=indexing
              i -> [w1004]
              n519 = case shown="5" w1004 {
                tunnel: w1003 -> [w1005 w1006 w1007 w1008 w1009 w1010]
                frame #0 {
                  n520 = local write "Roll Smoothing"(w1005) -> ()
                }
                frame #1 {
                  n521 = local write "Pitch Smoothing"(w1006) -> ()
                }
                frame #2 {
                  n522 = local write "Yaw  Smoothing"(w1007) -> ()
                }
                frame #3 {
                  n523 = local write "Throttle Smoothing"(w1008) -> ()
                }
                frame #4 {
                  n524 = local write "Mode  Smoothing"(w1009) -> ()
                }
                frame #5 {
                  n525 = local write "Aux  Smoothing"(w1010) -> ()
                }
              }
            }
          }
        }
        n526 = Bundle By Name(cluster=w965, "Error"=w964) -> (w963:T11)
      }
      frame #40 {
        n527 = Unbundle By Name(w1013) -> ("COMport"=w1014:refnum<visa-resource-name>, "Connected"=w1016:bool, "Error"=w1015:errorcluster)
        n528 = case shown="True" w1016 {
          tunnel: w1015 -> [w1017 w1019]
          tunnel: w1014 -> [_ w1022]
          tunnel: [w1017 w1026] -> w1011
          frame #0 {
          }
          frame #1 {
            w1018 = 0
            n529 = VISA Write(VISA resource name=w1022, write buffer="X", error in (no error)=w1019) -> (VISA resource name out=w1024:refnum<visa-resource-name>, error out=w1023:errorcluster)  [unwired: 1 out]
            n530 = call "Time Delay11"() -> ()  [unwired: 2 in, 10 out]
            n531 = VISA Flush I/O Buffer(VISA resource name=w1024, error in (no error)=w1023) -> (VISA resource name out=w1021:refnum<visa-resource-name>, error out=w1020:errorcluster)  [unwired: 1 in]
            n532 = property on="PlotSelection" class="Ring (strict)"("Value"=w1018) -> ()  [unwired: 2 in, 2 out]
            n533 = property on="GUI" class="TabCtl (strict)"("Val(Sgnl)"=w1018) -> ()  [unwired: 2 in, 2 out]
            n534 = Build Array("ProportionalRollLevel", "IntegralRollLevel", "DerivativeRollLevel", "ProportionalPitchLevel", "IntegralPitchLevel", "DerivativePitchLevel") -> (w1046:dbl[])
            n535 = call "WriteEEPROM.vi"("Query"="F", "Data"=w1046, "Command"="E", "error in"=w1020, "Skip"=TRUE, "VISA resource name"=w1021) -> ("error out"=w1049:errorcluster, "Checked Data"=w1037:dbl[], "Write Successful"=w1051:bool, "VISA resource name out"=w1050:refnum<visa-resource-name>)  [unwired: 1 in, 1 out]
            n536 = Index Array(array=w1037) -> (element #1=w1036:dbl, element #2=w1035:dbl, element #3=w1034:dbl, element #4=w1033:dbl, element #5=w1032:dbl, element #6=w1031:dbl)  [unwired: 6 in]
            n537 = local write "ProportionalRollLevel"(w1036) -> ()
            n538 = local write "IntegralRollLevel"(w1035) -> ()
            n539 = local write "DerivativeRollLevel"(w1034) -> ()
            n540 = local write "ProportionalPitchLevel"(w1033) -> ()